vi "Detector Test Program.vi"() -> ()   [LabVIEW 2020]
uses:
  RIMAS Detector Server Config.ctl
  RIMAS Observation Config.ctl
  RIMAS Detector Config.ctl
panel:
  out "FITS file acquired":path
  out "Image YJ raw frame":sgl[][](graph)
  out "Image HK raw frame":sgl[][](graph)
  in  "Detector Config":T1={"Detector"=0, "Offsets 0"=[0, 0, 0, 0, 0, 0, 0, 0, 0, 0, 0, 0, 0, 0, 0, 0, 0, 0, 0, 0, 0, 0, 0, 0, 0, 0, 0, 0, 0, 0, 0, 0], "Detector Computer"={"Machine"="192.168.121.11", "Password"="", "FITS File Path"="", "Port"=44444, "Header Path"="", "Simulate"=FALSE}, "FITS hdr template0"=path "", "FITS hdr template1"=path "", "FITS Data File Path"=path "", "FITS Detector Settings"={"Exp Time Short"=0.0, "# of Frames"=0.0, "Exp Time Long"=0.0, "# of Groups"=0.0, "Object Name"="", "Object"="", "Obs Type"="", "Image Type"="", "Observer"="", "Observer Affiliation"=""}, "Offsets 1"=[0, 0, 0, 0, 0, 0, 0, 0, 0, 0, 0, 0, 0, 0, 0, 0, 0, 0, 0, 0, 0, 0, 0, 0, 0, 0, 0, 0, 0, 0, 0, 0], "Sim Folder"=path ""} {"Offsets 1" format="%04x"; "Offsets 0" format="%04x"; "Detector" items=["0", "1", "2"]}
  # "sec"
  # "sec"
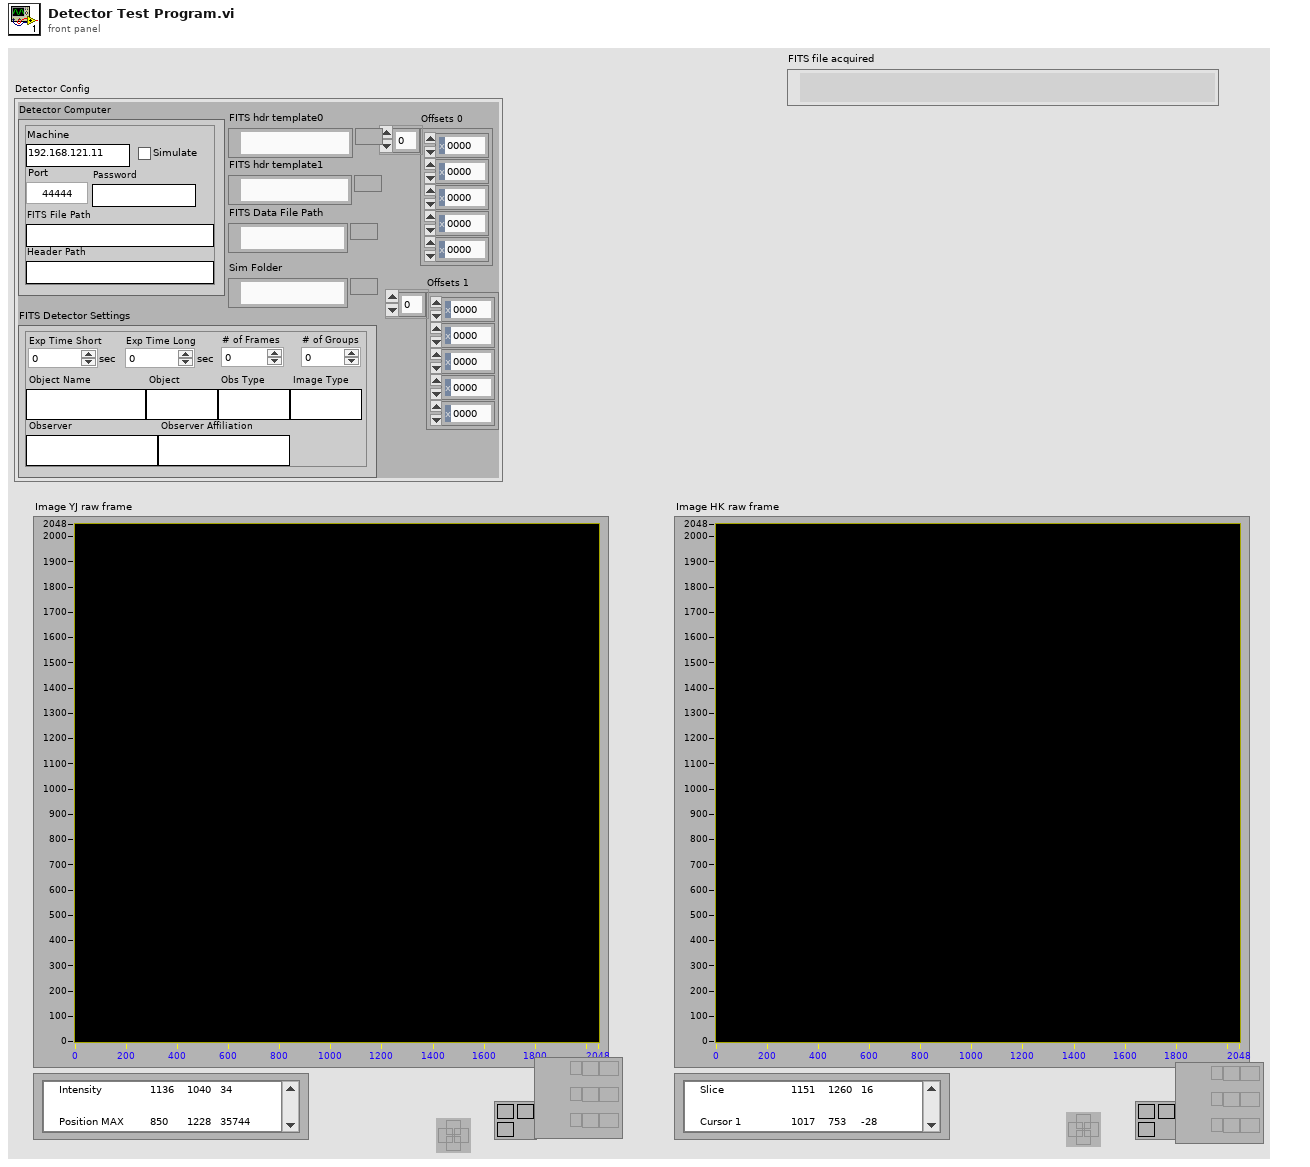
[diagram p1: front panel]
types:
  T1 = typedef "RIMAS Detector Config.ctl" = cluster{"Detector":u16, "Offsets 0":u16[], "Detector Computer":T2, "FITS hdr template0":path, "FITS hdr template1":path, "FITS Data File Path":path, "FITS Detector Settings":T3, "Offsets 1":u16[], "Sim Folder":path}
  T2 = typedef "RIMAS Detector Server Config.ctl" = cluster{"Machine":string, "Password":string, "FITS File Path":string, "Port":u16, "Header Path":string, "Simulate":bool}
  T3 = typedef "RIMAS Observation Config.ctl" = cluster{"Exp Time Short":dbl, "# of Frames":dbl, "Exp Time Long":dbl, "# of Groups":dbl, "Object Name":string, "Object":string, "Obs Type":string, "Image Type":string, "Observer":string, "Observer Affiliation":string}
  T4 = typedef "Detector Class.lvclass/Detector Image typedef cluster.ctl" = cluster{"Image":dbl[][], "Frame number":i32, "Detector #":u16, "FITS file acquired":path, "File size":i64}
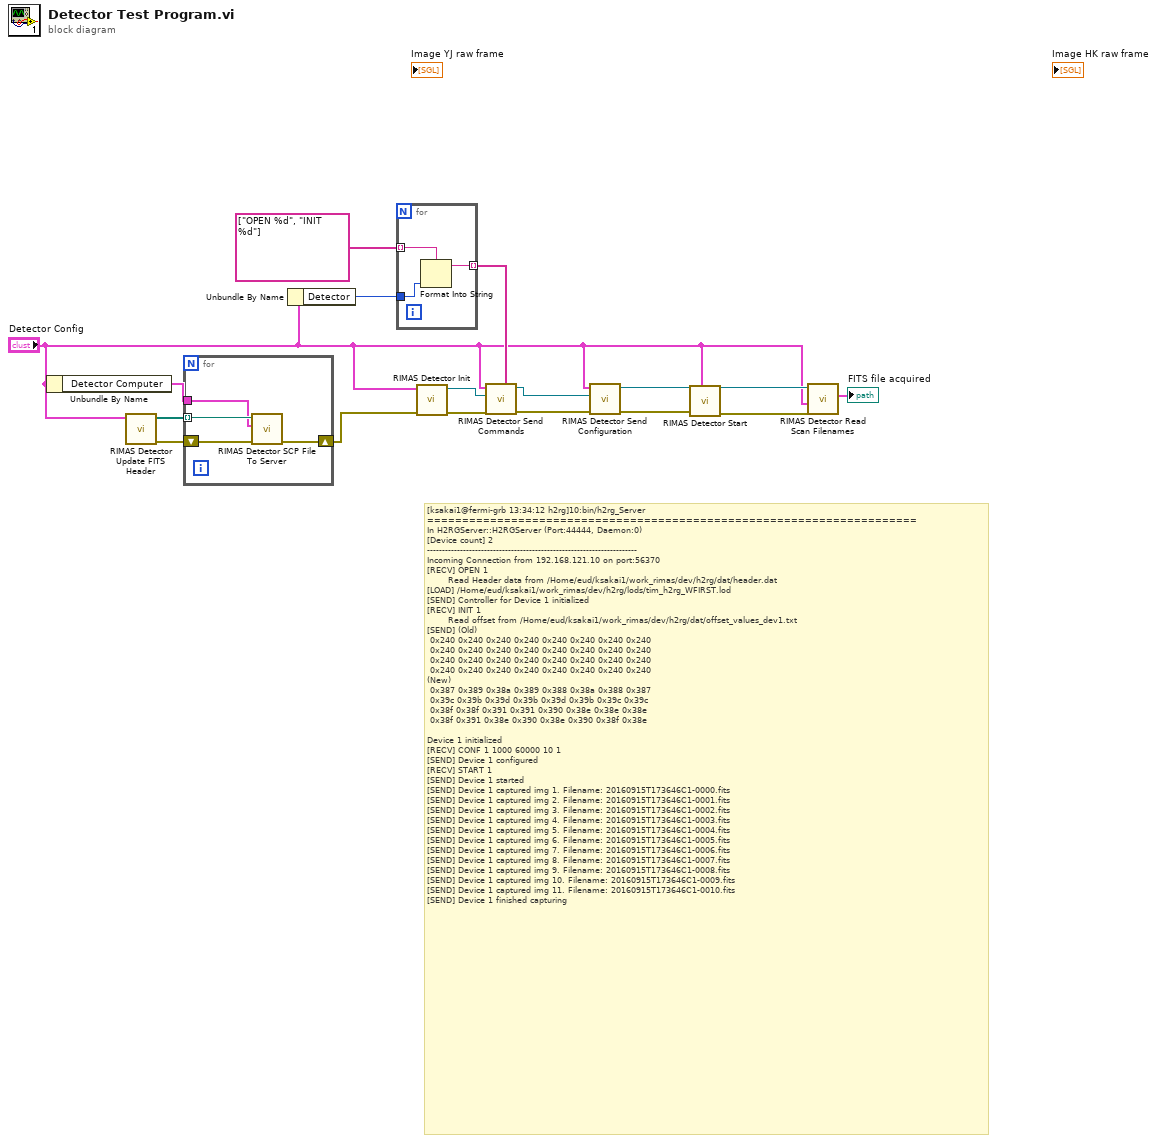
[diagram p0: block diagram]
diagram:
  # "[ksakai1@fermi-grb 13:34:12 h2rg]10:bin/h2rg_Server\n======================================================================\nIn H2RGServer::H2RGServer (Port:44444, Daemon:0)\n[Device count] 2\n----------------------------------------------------------------------\nIncoming Connection from 192.168.121.10 on port:56370\n[RECV] OPEN 1\n       Read Header data from /Home/eud/ksakai1/work_rimas/dev/h2rg/dat/header.dat\n[LOAD] /Home/eud/ksakai1/work_rimas/dev/h2rg/lods/tim_h2rg_WFIRST.lod\n[SEND] Controller for Device 1 initialized\n[RECV] INIT 1\n       Read offset from /Home/eud/ksakai1/work_rimas/dev/h2rg/dat/offset_values_dev1.txt\n[SEND] (Old)\n 0x240 0x240 0x240 0x240 0x240 0x240 0x240 0x240\n 0x240 0x240 0x240 0x240 0x240 0x240 0x240 0x240\n 0x240 0x240 0x240 0x240 0x240 0x240 0x240 0x240\n 0x240 0x240 0x240 0x240 0x240 0x240 0x240 0x240\n(New)\n 0x387 0x389 0x38a 0x389 0x388 0x38a 0x388 0x387\n 0x39c 0x39b 0x39d 0x39b 0x39d 0x39b 0x39c 0x39c\n 0x38f 0x38f 0x391 0x391 0x390 0x38e 0x38e 0x38e\n 0x38f 0x391 0x38e 0x390 0x38e 0x390 0x38f 0x38e\n\nDevice 1 initialized\n[RECV] CONF 1 1000 60000 10 1\n[SEND] Device 1 configured\n[RECV] START 1\n[SEND] Device 1 started\n[SEND] Device 1 captured img 1. Filename: 20160915T173646C1-0000.fits\n[SEND] Device 1 captured img 2. Filename: 20160915T173646C1-0001.fits\n[SEND] Device 1 captured img 3. Filename: 20160915T173646C1-0002.fits\n[SEND] Device 1 captured img 4. Filename: 20160915T173646C1-0003.fits\n[SEND] Device 1 captured img 5. Filename: 20160915T173646C1-0004.fits\n[SEND] Device 1 captured img 6. Filename: 20160915T173646C1-0005.fits\n[SEND] Device 1 captured img 7. Filename: 20160915T173646C1-0006.fits\n[SEND] Device 1 captured img 8. Filename: 20160915T173646C1-0007.fits\n[SEND] Device 1 captured img 9. Filename: 20160915T173646C1-0008.fits\n[SEND] Device 1 captured img 10. Filename: 20160915T173646C1-0009.fits\n[SEND] Device 1 captured img 11. Filename: 20160915T173646C1-0010.fits\n[SEND] Device 1 finished capturing"
  n1 = Unbundle By Name("Detector Config") -> ("Detector Computer"=w14:T2)
  n2 = call "RIMAS Detector Update FITS Header.vi"("Detector Config"="Detector Config") -> ("Error Out"=w15:errorcluster, "Files"=w16:path[])  [unwired: 9 in]
  n3 = for {
    tunnel: w16 -> [w21] mode=indexing
    tunnel: w14 -> [w20]
    shift-right: [w18] -> w13
    shift-left: w15 -> [w19]
    n4 = call "RIMAS Detector SCP File To Server.vi"("Error In"=w19, "Detector Computer"=w20, "Local File Path"=w21) -> ("Error Out"=w18:errorcluster)  [unwired: 7 in, 1 out]
  }
  n5 = Unbundle By Name("Detector Config") -> ("Detector"=w10:u16)
  n6 = for {
    tunnel: string[] ["OPEN %d", "INIT %d"] ("Cmds") -> [w24] mode=indexing
    tunnel: w10 -> [w23]
    tunnel: [w22] -> w9 mode=indexing
    n7 = Format Into String(format string=w24, w23) -> (resulting string=w22:string)  [unwired: 2 in, 1 out]
  }
  n8 = call "RIMAS Detector Init.vi"("Error In"=w13, "Detector Config"="Detector Config") -> ("Error Out"=w8:errorcluster, "Detector Ref"=w12:refnum<k5>)  [unwired: 7 in, 1 out]
  n9 = call "RIMAS Detector Send Commands.vi"("Cmds"=w9, "Error In"=w8, "Detector Ref in"=w12, "Detector Config"="Detector Config") -> ("Error Out"=w5:errorcluster, "Detector Ref"=w7:refnum<k5>)  [unwired: 4 in, 2 out]
  n10 = call "RIMAS Detector Send Configuration.vi"("Error In"=w5, "Detector Ref in"=w7, "Detector Config"="Detector Config") -> ("Error Out"=w4:errorcluster, "Detector Ref"=w3:refnum<k5>)  [unwired: 4 in, 3 out]
  n11 = call "RIMAS Detector Start.vi"(7:"Detector Config", "Error In"=w4, "Detector Ref in"=w3) -> ("Error Out"=w2:errorcluster, "Detector Ref out"=w17:refnum<k5>)  [unwired: 7 in]
  n12 = call "RIMAS Detector Read Scan Filenames.vi"("Error In"=w2, "Detector Config"="Detector Config", "Detector Ref"=w17) -> ("Image Data"=→"FITS file acquired":T4)  [unwired: 3 in, 5 out]
